vi "snake server.vi"() -> ()   [LabVIEW 2015]
uses:
  <vilib>/event_ctls.llb/eventvkey.ctl
  <vilib>/picture/picture.llb/Draw True-Color Pixmap.vi
panel:
  out "score 2":i32
  in  "path":path
  out "y":i32
  out "x":i32
  out "food y":i32
  out "food x":i32
  out "x .and. y?":bool
  out "Numeric":i32
  out "2D Picture":picture
  out "score":i32
  out "VKey":T1
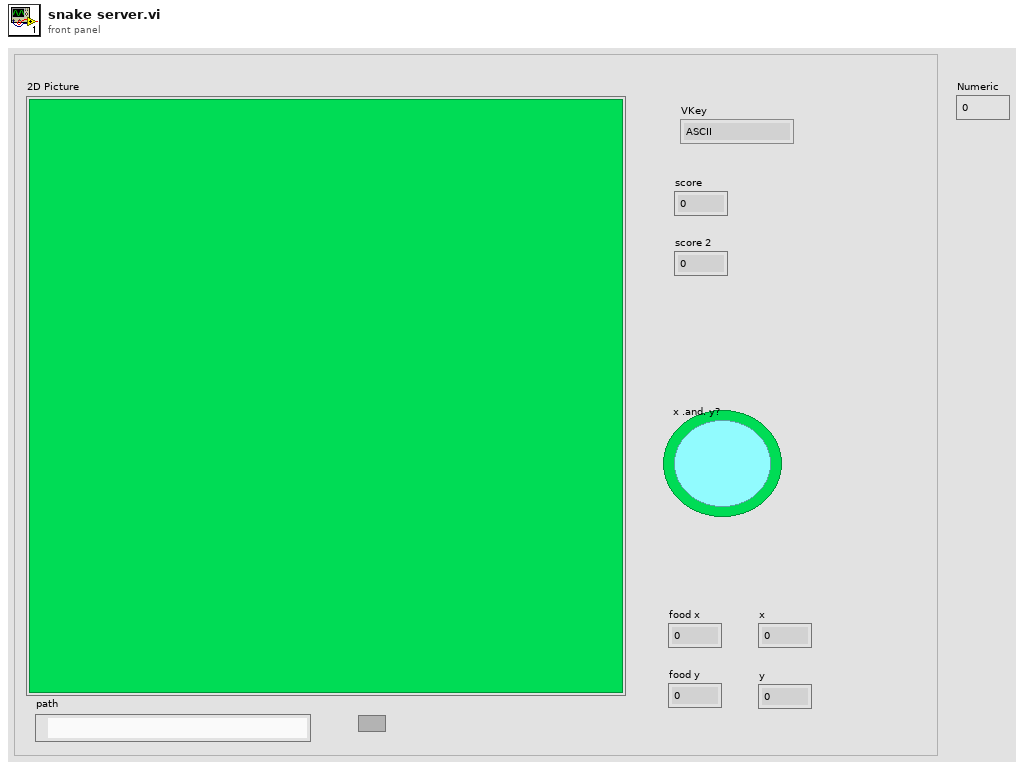
[diagram p1: front panel]
types:
  T1 = typedef "eventvkey.ctl" = enum16{"ASCII", "Enter", "Return", "Shift", "Ctrl", "Alt", "Cmd", "Opt", "Caps", "NumLock", "Clear", "Break", "Up", "Down", "Left", "Right", "Insert", "Delete", "Home", "End", "PageUp", "PageDown", "Escape", "Help", "Pause", "ScrollLock", "F1", "F2", "F3", "F4", "F5", "F6", "F7", "F8", "F9", "F10", "F11", "F12", "F13", "F14", "F15", "F16", "F17", "F18", "F19", "F20", "F21", "F22", "F23", "F24", "Play", "VolumeUp", "VolumeDown", "Mute", "Two Byte Char"}
  T2 = enum16{"Read", "Write", "ReadWrite", "BufferedRead", "BufferedReadWrite"}
  T3 = cluster{"food x":i32, "food y":i32, "direction":string, "snake x":i32[], "snake y":i32[], "food":bool}
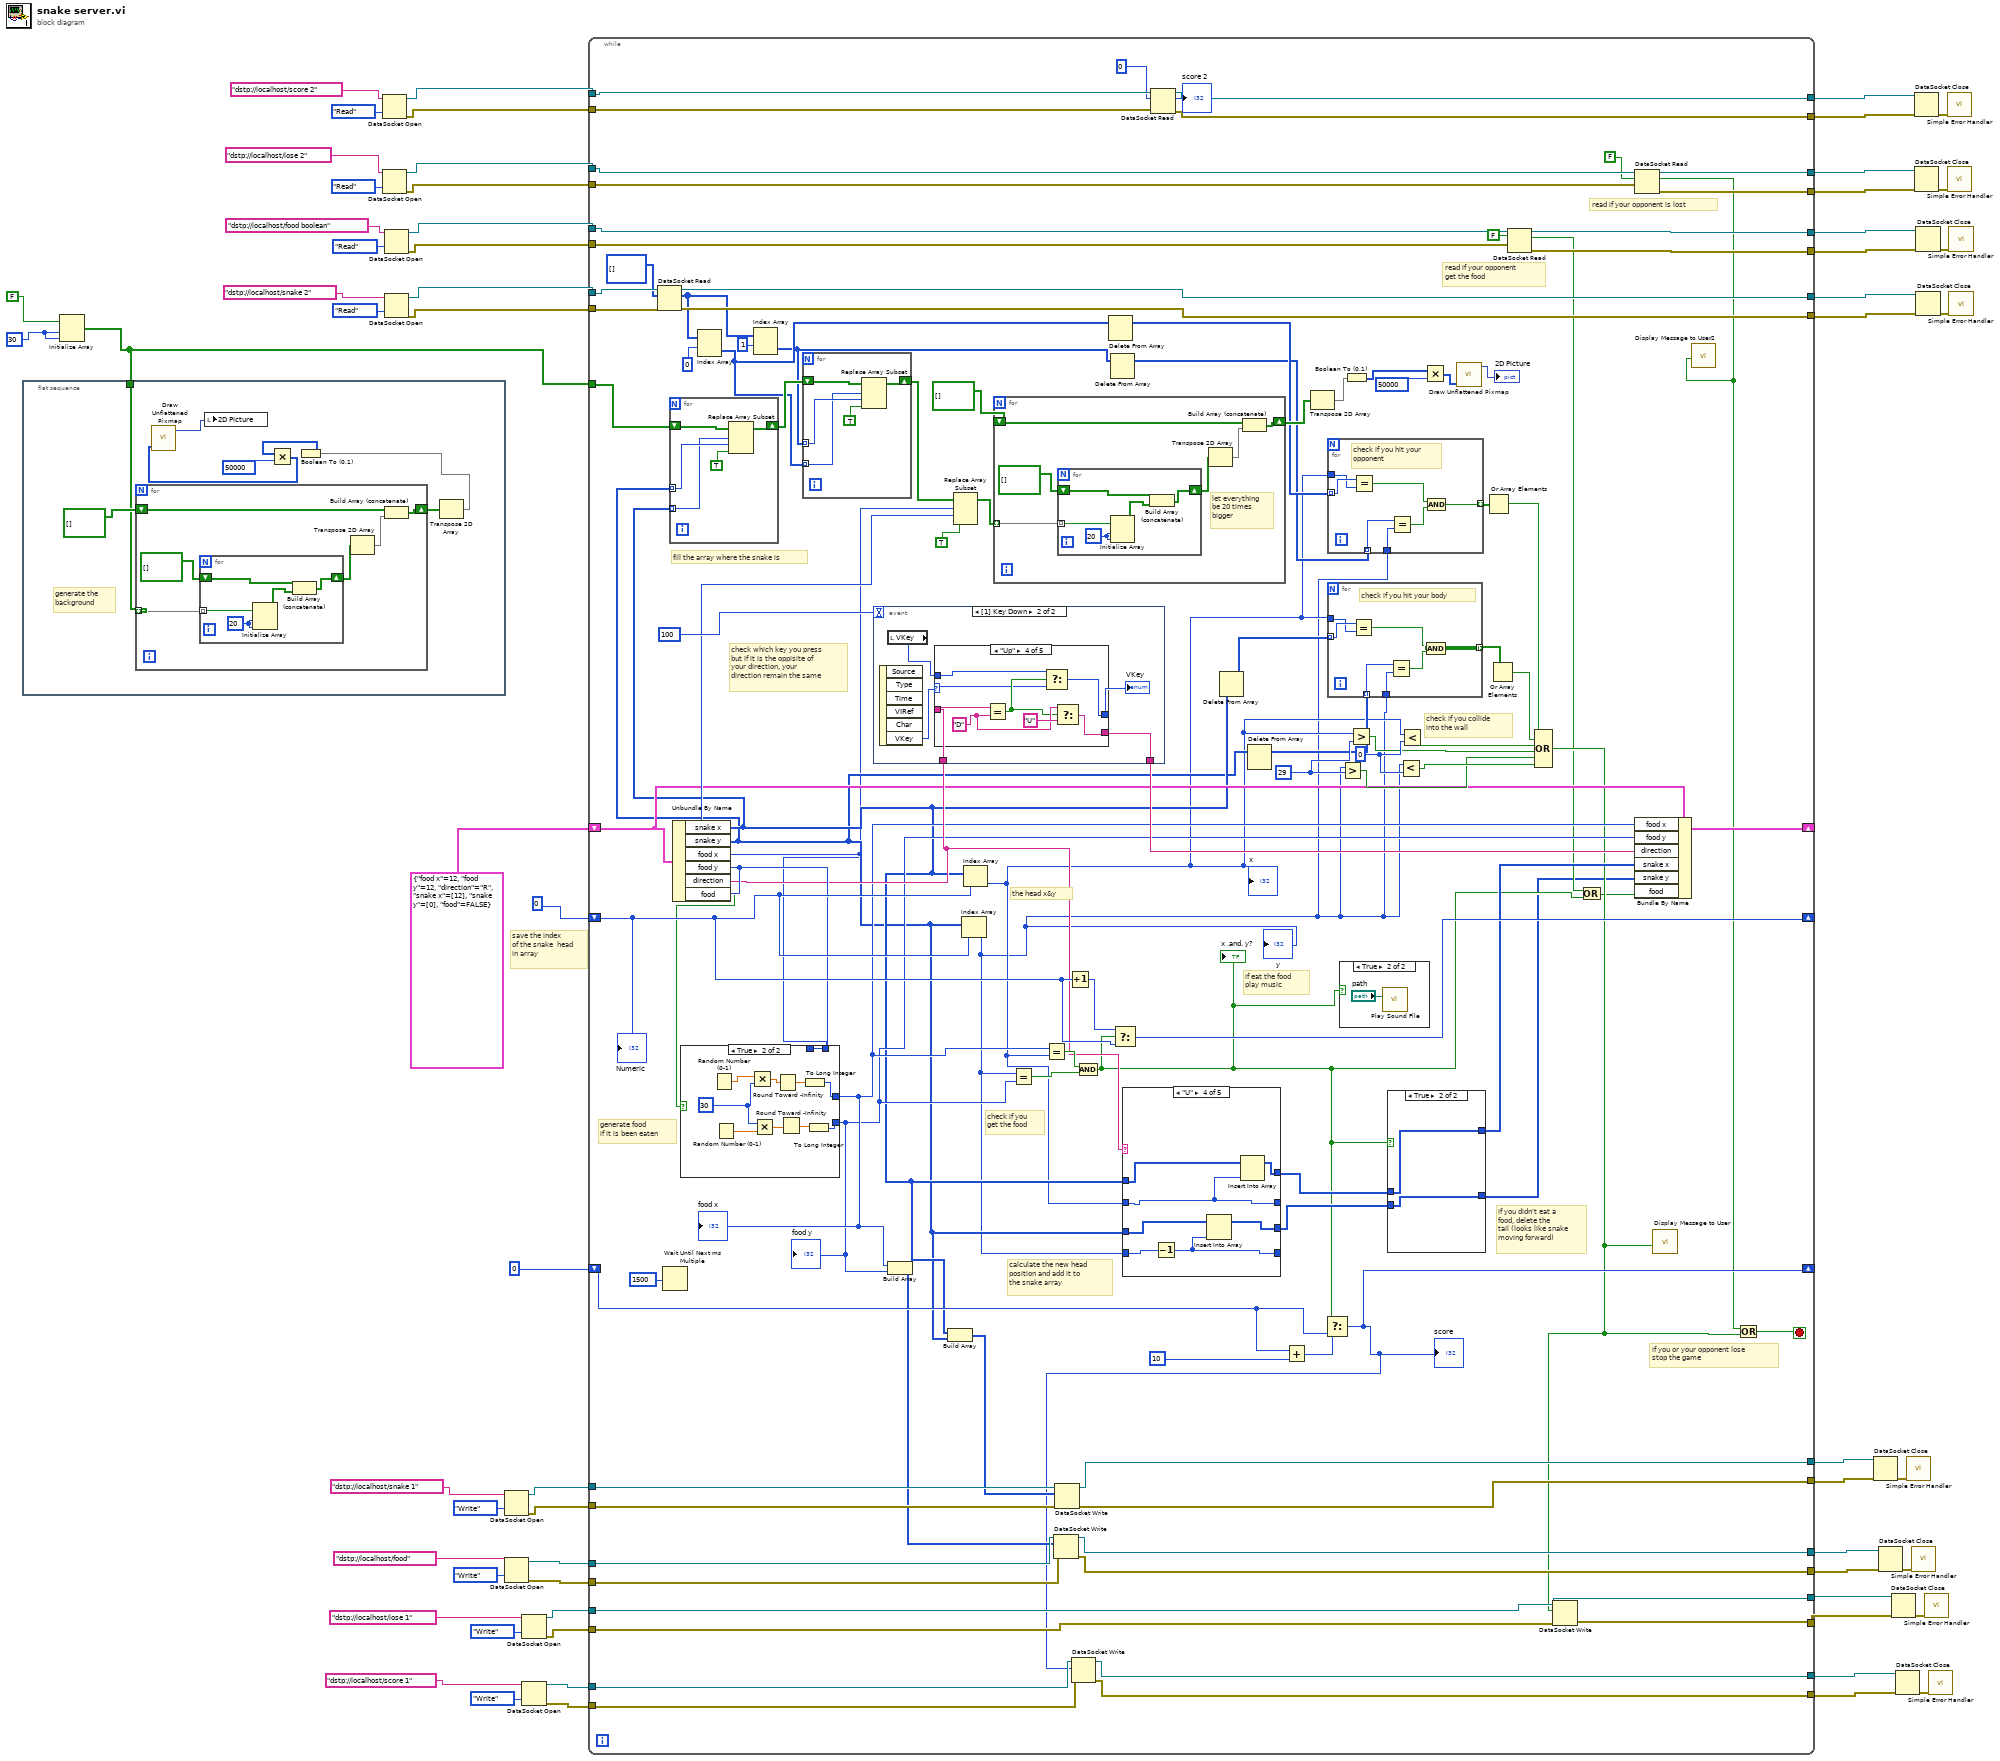
[diagram p0: block diagram]
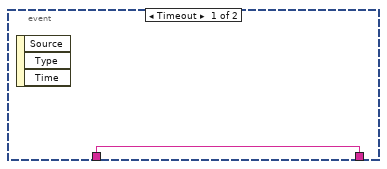
[diagram p3: hidden frame]
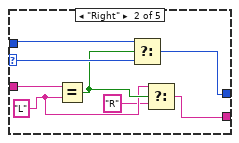
[diagram p5: hidden frame]
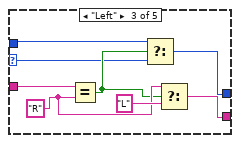
[diagram p6: hidden frame]
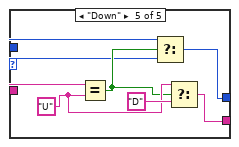
[diagram p7: hidden frame]
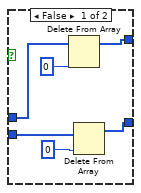
[diagram p8: hidden frame]
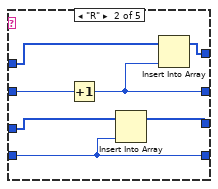
[diagram p10: hidden frame]
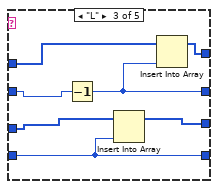
[diagram p11: hidden frame]
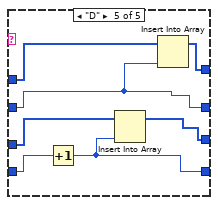
[diagram p12: hidden frame]
diagram:
  w59 = 30
  # "save the index\nof the snake  head in array"
  n1 = flat-sequence {
    tunnel: w57 -> [w63]
    frame #0 {
      # "generate the \nbackground"
      n2 = for {
        tunnel: w63 -> [w76] mode=indexing
        shift-right: [w71] -> w69
        shift-left: bool[][] [] -> [w72]
        n3 = for {
          tunnel: w76 -> [w81] mode=indexing
          shift-right: [w77] -> w74
          shift-left: bool[][] [] -> [w78]
          w80 = 20
          n4 = Initialize Array(w81, w80, w80) -> (w79:bool[][])
          n5 = Build Array (concatenate)(w78, w79) -> (w77:bool[][])
        }
        n6 = Transpose 2D Array(2D array=w74) -> (transposed array=w73:bool[][])
        n7 = Build Array (concatenate)(w72, w73) -> (w71:bool[][])
      }
      n8 = Transpose 2D Array(2D array=w69) -> (transposed array=w68:bool[][])
      n9 = Boolean To (0,1)(Boolean=w68) -> (0, 1=w67:i16[][])
      n10 = Multiply(x=w67, y=50000) -> (x*y=w65:i32[][])
      n11 = call-poly <vilib>:"Draw Unflattened Pixmap.vi"("data (RGB format)"=w65) -> ("new picture"=w64:picture)  [unwired: 8 in]
      n12 = local write "2D Picture"(w64) -> ()
    }
  }
  n13 = Initialize Array(FALSE, w59, w59) -> (w57:bool[][])
  n14 = DataSocket Open(10:T2."Read" ("mode"), 11:"dstp://localhost/score 2") -> (0:w11:errorcluster, 3:w12:refnum<k13>)  [unwired: 2 in]
  n15 = DataSocket Open(10:T2."Read" ("mode"), 11:"dstp://localhost/lose 2") -> (0:w20:errorcluster, 3:w19:refnum<k13>)  [unwired: 2 in]
  n16 = DataSocket Open(10:T2."Read" ("mode"), 11:"dstp://localhost/food boolean") -> (0:w22:errorcluster, 3:w23:refnum<k13>)  [unwired: 2 in]
  n17 = DataSocket Open(10:T2."Read" ("mode"), 11:"dstp://localhost/snake 2") -> (0:w43:errorcluster, 3:w42:refnum<k13>)  [unwired: 2 in]
  n18 = DataSocket Open(10:T2."Write" ("mode"), 11:"dstp://localhost/snake 1" ("URL")) -> (0:w55:errorcluster, 3:w56:refnum<k13>)  [unwired: 2 in]
  n19 = DataSocket Open(10:T2."Write" ("mode"), 11:"dstp://localhost/food" ("URL")) -> (0:w48:errorcluster, 3:w49:refnum<k13>)  [unwired: 2 in]
  n20 = DataSocket Open(10:T2."Write" ("mode"), 11:"dstp://localhost/lose 1" ("URL")) -> (0:w28:errorcluster, 3:w27:refnum<k13>)  [unwired: 2 in]
  n21 = DataSocket Open(10:T2."Write" ("mode"), 11:"dstp://localhost/score 1" ("URL")) -> (0:w35:errorcluster, 3:w34:refnum<k13>)  [unwired: 2 in]
  n22 = while {
    shift-right: [w185] -> _
    shift-left: T3 {"food x"=12, "food y"=12, "direction"="R", "snake x"=[12], "snake y"=[0], "food"=FALSE} -> [w128]
    shift-right: [w181] -> _
    shift-left: 0 -> [w179]
    shift-right: [w121] -> _
    shift-left: 0 -> [w154]
    tunnel: w57 -> [w162]
    tunnel: w56 -> [w150]
    tunnel: w55 -> [w149]
    tunnel: [w148] -> w53
    tunnel: [w147] -> w52
    tunnel: w49 -> [w145]
    tunnel: w48 -> [w144]
    tunnel: [w143] -> w46
    tunnel: [w142] -> w45
    tunnel: w43 -> [w140]
    tunnel: w42 -> [w141]
    tunnel: [w139] -> w40
    tunnel: [w138] -> w39
    tunnel: w27 -> [w129]
    tunnel: w28 -> [w130]
    tunnel: [w131] -> w30
    tunnel: [w132] -> w31
    tunnel: w34 -> [w133]
    tunnel: w35 -> [w134]
    tunnel: [w135] -> w37
    tunnel: [w136] -> w38
    tunnel: w22 -> [w118]
    tunnel: w23 -> [w117]
    tunnel: [w119] -> w25
    tunnel: [w120] -> w26
    tunnel: w20 -> [w115]
    tunnel: w19 -> [w116]
    tunnel: [w114] -> w17
    tunnel: [w113] -> w16
    tunnel: w11 -> [w110]
    tunnel: w12 -> [w109]
    tunnel: [w111] -> w14
    tunnel: [w112] -> w15
    stop <- w104 stop-if-true
    w172 = 29
    w171 = 0
    # "fill the array where the snake is"
    # "read if your opponent \nget the food"
    # "read if your opponent is lost"
    # "if you or your opponent lose\nstop the game"
    # "check if you collide\ninto the wall"
    # "check which key you press\nbut if it is the oppisite of \nyour direction, your\ndirection remain the same"
    # "if you didn't eat a\nfood, delete the \ntail (looks like snake\nmoving forward)"
    # "calculate the new head\nposition and add it to\nthe snake array"
    # "check if you\nget the food"
    # "if eat the food\nplay music"
    # "the head x&y"
    # "generate food\nif it is been eaten"
    n23 = DataSocket Read(8:w140, 10:i32[][] [], 11:w141) -> (0:w138:errorcluster, 2:w95:i32[][], 3:w139:refnum<k13>)  [unwired: 2 in, 4 out]
    n24 = Wait Until Next ms Multiple(millisecond multiple=u32 1500) -> ()  [unwired: 1 out]
    n25 = Unbundle By Name(w128) -> ("snake x"=w124:i32[], "snake y"=w123:i32[], "food x"=w99:i32, "food y"=w155:i32, "direction"=w146:string, "food"=w137:bool)
    n26 = for {
      tunnel: w124 -> [w210] mode=indexing
      tunnel: w123 -> [w211] mode=indexing
      shift-right: [w212] -> w98
      shift-left: w162 -> [w214]
      n27 = Replace Array Subset(array=w214, new element=TRUE, index (row)=w210, index (col)=w211) -> (w212:bool[][])
    }
    n28 = case shown="True" w137 {
      tunnel: w99 -> [w302 _]
      tunnel: w155 -> [w303 _]
      tunnel: [w303 w304] -> w126
      tunnel: [w302 w306] -> w127
      frame False {
      }
      frame True {
        w312 = 30
        n29 = Random Number (0-1)() -> (number: 0 to 1=w310:dbl)
        n30 = Random Number (0-1)() -> (number: 0 to 1=w311:dbl)
        n31 = Multiply(x=w310, y=w312) -> (x*y=w309:dbl)
        n32 = Multiply(x=w312, y=w311) -> (x*y=w308:dbl)
        n33 = Round Toward -Infinity(1:w309) -> (0:w307:dbl)
        n34 = Round Toward -Infinity(1:w308) -> (0:w305:dbl)
        n35 = To Long Integer(number=w307) -> (32bit integer=w306:i32)
        n36 = To Long Integer(number=w305) -> (32bit integer=w304:i32)
      }
    }
    "food x" <- w127
    "food y" <- w126
    n37 = Index Array(array=w95, index (row)=0) -> (element=w92:i32[])  [unwired: 1 in]
    n38 = Index Array(array=w95, index (row)=1) -> (element=w91:i32[])  [unwired: 1 in]
    n39 = for {
      tunnel: w92 -> [w194] mode=indexing
      tunnel: w91 -> [w195] mode=indexing
      shift-right: [w196] -> w97
      shift-left: w98 -> [w198]
      n40 = Replace Array Subset(array=w198, new element=TRUE, index (row)=w194, index (col)=w195) -> (w196:bool[][])
    }
    n41 = event shown="[1] Key Down" {
      selector: _ -> [_ _]
      dyn-events: _ -> [_ _]
      timeout: 100 -> [_ _]
      tunnel: w146 -> [w222 w224]
      tunnel: [w222 w223] -> w177
      event Timeout {
        n42 = event-data() -> ()  [unwired: 1 in, 3 out]
      }
      event Key Down {
        n43 = event-data() -> ("VKey"=w227:T1)  [unwired: 1 in, 5 out]
        n44 = local read "VKey"() -> (w225:T1)
        n45 = case shown="\"Up\"" w227 {
          selector: w227 -> [_ w235 w241 w247 w254]
          tunnel: [w229 w234 w238 w250 w258] -> w226
          tunnel: w225 -> [w229 w236 w242 w248 w255]
          tunnel: w224 -> [w228 w237 w240 w246 w256]
          tunnel: [w228 w232 w239 w249 w257] -> w223
          frame "ASCII", Default {
          }
          frame "Right" {
            w231 = "L"
            n46 = Equal?(x=w237, y=w231) -> (x = y?=w233:bool)
            n47 = Select(t=w236, s=w233, f=w235) -> (s? t:f=w234:T1)
            n48 = Select(t=w231, s=w233, f="R") -> (s? t:f=w232:string)
          }
          frame "Left" {
            w244 = "R"
            n49 = Equal?(x=w240, y=w244) -> (x = y?=w243:bool)
            n50 = Select(t=w242, s=w243, f=w241) -> (s? t:f=w238:T1)
            n51 = Select(t=w244, s=w243, f="L") -> (s? t:f=w239:string)
          }
          frame "Up" {
            w252 = "D"
            n52 = Equal?(x=w246, y=w252) -> (x = y?=w251:bool)
            n53 = Select(t=w248, s=w251, f=w247) -> (s? t:f=w250:T1)
            n54 = Select(t=w252, s=w251, f="U") -> (s? t:f=w249:string)
          }
          frame "Down" {
            w260 = "U"
            n55 = Equal?(x=w256, y=w260) -> (x = y?=w259:bool)
            n56 = Select(t=w255, s=w259, f=w254) -> (s? t:f=w258:T1)
            n57 = Select(t=w260, s=w259, f="D") -> (s? t:f=w257:string)
          }
        }
        "VKey" <- w226
      }
    }
    n58 = Build Array(w127, w126) -> (w125:i32[])
    n59 = Build Array(w124, w123) -> (w122:i32[][])
    n60 = Replace Array Subset(array=w97, new element=TRUE, index (row)=w99, index (col)=w155) -> (w100:bool[][])
    n61 = Index Array(array=w123, index=w179) -> (element=w87:i32)
    "y" <- w87
    n62 = Index Array(array=w124, index=w179) -> (element=w88:i32)
    "x" <- w88
    n63 = for {
      tunnel: w100 -> [w204] mode=indexing
      shift-right: [w199] -> w152
      shift-left: bool[][] [] -> [w200]
      # "let everything\nbe 20 times \nbigger"
      n64 = for {
        tunnel: w204 -> [w209] mode=indexing
        shift-right: [w205] -> w202
        shift-left: bool[][] [] -> [w206]
        w208 = 20
        n65 = Initialize Array(w209, w208, w208) -> (w207:bool[][])
        n66 = Build Array (concatenate)(w206, w207) -> (w205:bool[][])
      }
      n67 = Transpose 2D Array(2D array=w202) -> (transposed array=w201:bool[][])
      n68 = Build Array (concatenate)(w200, w201) -> (w199:bool[][])
    }
    n69 = Equal?(x=w87, y=w126) -> (x = y?=w183:bool)
    n70 = Equal?(x=w127, y=w88) -> (x = y?=w182:bool)
    n71 = DataSocket Write(8:w144, 10:w125, 11:w145) -> (0:w142:errorcluster, 3:w143:refnum<k13>)  [unwired: 1 in, 1 out]
    n72 = DataSocket Write(8:w149, 10:w122, 11:w150) -> (0:w147:errorcluster, 3:w148:refnum<k13>)  [unwired: 1 in, 1 out]
    n73 = Increment(x=w179) -> (x+1=w180:i32)
    n74 = And(x=w182, y=w183) -> (x .and. y?=w84:bool)
    "x .and. y?" <- w84
    n75 = Delete From Array(array=w92) -> (array with subset deleted=w90:i32[])  [unwired: 2 in, 1 out]
    n76 = Delete From Array(array=w91) -> (array with subset deleted=w89:i32[])  [unwired: 2 in, 1 out]
    n77 = Select(t=w180, s=w84, f=w179) -> (s? t:f=w181:i32)
    n78 = case shown="\"U\"" w146 {
      tunnel: w124 -> [w273 w275 w286 w294 w298]
      tunnel: w123 -> [w271 w278 w284 w293 w300]
      tunnel: w88 -> [w272 w280 w285 w289 w299]
      tunnel: w87 -> [w270 w279 w283 w290 w301]
      tunnel: [w270 w279 w283 w288 w295] -> _
      tunnel: [w272 w276 w281 w289 w299] -> _
      tunnel: [w271 w277 w282 w292 w296] -> w176
      tunnel: [w273 w274 w287 w291 w297] -> w175
      frame "False", Default {
      }
      frame "R" {
        n79 = Increment(x=w280) -> (x+1=w276:i32)
        n80 = Insert Into Array(array=w278, new element=w279) -> (w277:i32[])  [unwired: 1 in]
        n81 = Insert Into Array(array=w275, new element=w276) -> (w274:i32[])  [unwired: 1 in]
      }
      frame "L" {
        n82 = Decrement(x=w285) -> (x-1=w281:i32)
        n83 = Insert Into Array(array=w284, new element=w283) -> (w282:i32[])  [unwired: 1 in]
        n84 = Insert Into Array(array=w286, new element=w281) -> (w287:i32[])  [unwired: 1 in]
      }
      frame "U" {
        n85 = Decrement(x=w290) -> (x-1=w288:i32)
        n86 = Insert Into Array(array=w293, new element=w288) -> (w292:i32[])  [unwired: 1 in]
        n87 = Insert Into Array(array=w294, new element=w289) -> (w291:i32[])  [unwired: 1 in]
      }
      frame "D" {
        n88 = Increment(x=w301) -> (x+1=w295:i32)
        n89 = Insert Into Array(array=w300, new element=w295) -> (w296:i32[])  [unwired: 1 in]
        n90 = Insert Into Array(array=w298, new element=w299) -> (w297:i32[])  [unwired: 1 in]
      }
    }
    n91 = DataSocket Read(8:w110, 10:0, 11:w109) -> (0:w112:errorcluster, 2:→"score 2":i32, 3:w111:refnum<k13>)  [unwired: 2 in, 4 out]
    n92 = Delete From Array(array=w124) -> (array with subset deleted=w165:i32[])  [unwired: 2 in, 1 out]
    n93 = Delete From Array(array=w123) -> (array with subset deleted=w164:i32[])  [unwired: 2 in, 1 out]
    n94 = Add(x=w154, y=10) -> (x+y=w163:i32)
    n95 = Transpose 2D Array(2D array=w152) -> (transposed array=w151:bool[][])
    n96 = Select(t=w163, s=w84, f=w154) -> (s? t:f=w121:i32)
    "score" <- w121
    n97 = DataSocket Write(8:w134, 10:w121, 11:w133) -> (0:w136:errorcluster, 3:w135:refnum<k13>)  [unwired: 1 in, 1 out]
    n98 = for {
      tunnel: w165 -> [w221] mode=indexing
      tunnel: w164 -> [w218] mode=indexing
      tunnel: w88 -> [w220]
      tunnel: w87 -> [w219]
      tunnel: [w215] -> w173 mode=indexing
      # "check if you hit your body"
      n99 = Equal?(x=w221, y=w220) -> (x = y?=w216:bool)
      n100 = Equal?(x=w218, y=w219) -> (x = y?=w217:bool)
      n101 = And(x=w216, y=w217) -> (x .and. y?=w215:bool)
    }
    n102 = for {
      tunnel: w90 -> [w193] mode=indexing
      tunnel: w89 -> [w190] mode=indexing
      tunnel: w88 -> [w192]
      tunnel: w87 -> [w191]
      tunnel: [w187] -> w86 mode=indexing
      # "check if you hit your\nopponent"
      n103 = Equal?(x=w193, y=w192) -> (x = y?=w188:bool)
      n104 = Equal?(x=w190, y=w191) -> (x = y?=w189:bool)
      n105 = And(x=w188, y=w189) -> (x .and. y?=w187:bool)
    }
    n106 = case shown="True" w84 {
      frame False {
      }
      frame True {
        n107 = call <vilib>:"Play Sound File.vi"("path"="path") -> ()  [unwired: 9 in, 2 out]
      }
    }
    n108 = Greater?(x=w87, y=w172) -> (0:w166:bool)
    n109 = Boolean To (0,1)(Boolean=w151) -> (0, 1=w159:i16[][])
    n110 = Greater?(x=w88, y=w172) -> (0:w168:bool)
    n111 = case shown="True" w84 {
      tunnel: w176 -> [w265 w268]
      tunnel: w175 -> [w264 w269]
      tunnel: [w263 w269] -> w174
      tunnel: [w262 w268] -> w82
      frame False {
        n112 = Delete From Array(array=w264, index=0) -> (array with subset deleted=w263:i32[])  [unwired: 1 in, 1 out]
        n113 = Delete From Array(array=w265, index=0) -> (array with subset deleted=w262:i32[])  [unwired: 1 in, 1 out]
      }
      frame True {
      }
    }
    n114 = Less?(x=w87, y=w171) -> (x < y?=w167:bool)
    n115 = Less?(x=w88, y=w171) -> (x < y?=w169:bool)
    n116 = Multiply(x=w159, y=50000) -> (x*y=w158:i32[][])
    n117 = call-poly <vilib>:"Draw Unflattened Pixmap.vi"("data (RGB format)"=w158) -> ("new picture"=→"2D Picture":picture)  [unwired: 8 in]
    n118 = Or Array Elements(Boolean array=w86) -> (logical OR=w85:bool)
    n119 = Or Array Elements(Boolean array=w173) -> (logical OR=w170:bool)
    n120 = DataSocket Read(8:w118, 10:FALSE, 11:w117) -> (0:w120:errorcluster, 2:w101:bool, 3:w119:refnum<k13>)  [unwired: 2 in, 4 out]
    n121 = Compound Arithmetic op=OR(w85, w170, w169, w168, w166, w167) -> (w105:bool)
    n122 = DataSocket Write(8:w130, 10:w105, 11:w129) -> (0:w132:errorcluster, 3:w131:refnum<k13>)  [unwired: 1 in, 1 out]
    n123 = Or(x=w101, y=w84) -> (x .or. y?=w102:bool)
    n124 = Bundle By Name(cluster=w128, "food x"=w127, "food y"=w126, "direction"=w177, "snake x"=w174, "snake y"=w82, "food"=w102) -> (w185:T3)
    n125 = DataSocket Read(8:w115, 10:FALSE, 11:w116) -> (0:w113:errorcluster, 2:w103:bool, 3:w114:refnum<k13>)  [unwired: 2 in, 4 out]
    n126 = call "Display Message to User"("Enable"=w105) -> ()  [unwired: 9 in, 2 out]
    n127 = call "Display Message to User2"("Enable"=w103) -> ()  [unwired: 9 in, 2 out]
    n128 = Or(x=w103, y=w105) -> (x .or. y?=w104:bool)
    "Numeric" <- w179
  }
  n129 = DataSocket Close(8:w52, 11:w53) -> (0:w51:errorcluster)  [unwired: 1 in, 1 out]
  n130 = DataSocket Close(8:w45, 11:w46) -> (0:w47:errorcluster)  [unwired: 1 in, 1 out]
  n131 = DataSocket Close(8:w31, 11:w30) -> (0:w32:errorcluster)  [unwired: 1 in, 1 out]
  n132 = DataSocket Close(8:w38, 11:w37) -> (0:w36:errorcluster)  [unwired: 1 in, 1 out]
  n133 = call <vilib>:"Simple Error Handler.vi"("error in (no error)"=w51) -> ()  [unwired: 4 in, 5 out]
  n134 = call <vilib>:"Simple Error Handler.vi"("error in (no error)"=w47) -> ()  [unwired: 4 in, 5 out]
  n135 = DataSocket Close(8:w15, 11:w14) -> (0:w13:errorcluster)  [unwired: 1 in, 1 out]
  n136 = DataSocket Close(8:w16, 11:w17) -> (0:w18:errorcluster)  [unwired: 1 in, 1 out]
  n137 = DataSocket Close(8:w26, 11:w25) -> (0:w24:errorcluster)  [unwired: 1 in, 1 out]
  n138 = DataSocket Close(8:w39, 11:w40) -> (0:w41:errorcluster)  [unwired: 1 in, 1 out]
  n139 = call <vilib>:"Simple Error Handler.vi"("error in (no error)"=w32) -> ()  [unwired: 4 in, 5 out]
  n140 = call <vilib>:"Simple Error Handler.vi"("error in (no error)"=w36) -> ()  [unwired: 4 in, 5 out]
  n141 = call <vilib>:"Simple Error Handler.vi"("error in (no error)"=w13) -> ()  [unwired: 4 in, 5 out]
  n142 = call <vilib>:"Simple Error Handler.vi"("error in (no error)"=w18) -> ()  [unwired: 4 in, 5 out]
  n143 = call <vilib>:"Simple Error Handler.vi"("error in (no error)"=w24) -> ()  [unwired: 4 in, 5 out]
  n144 = call <vilib>:"Simple Error Handler.vi"("error in (no error)"=w41) -> ()  [unwired: 4 in, 5 out]
